vi "TLB Native Dynamic Events ver 0.26b.vi"() -> ()   [LabVIEW 2018] (continued)
                      n634 = Enqueue Element(queue=w1888, element=w1886) -> (queue out=w1887:refnum<queue>)  [unwired: 2 in, 2 out]
                    }
                  }
                }
                n635 = Or(x=w1870, y=w1866) -> (x .or. y?=w1873:bool)
                n636 = Select(t=State_Type_Definitions,_for_0.26g_versions_and_later_2."True Stop" ("Enum"), s=w1866, f=State_Type_Definitions,_for_0.26g_versions_and_later_2."Task 8K: RAISE MY SWORD" ("Enum")) -> (s? t:f=w1868:T18)
                n637 = Select(t=w1868, s=w1873, f=State_Type_Definitions,_for_0.26g_versions_and_later_2."Task 8J: CLOSE CLAW" ("Enum")) -> (s? t:f=w1872:T18)
              }
              frame "Exit" {
                n638 = for {
                  shift-right: [w1895] -> w1892
                  shift-left: w1889 -> [w1896]
                  tunnel: string[] ["STOP", "RESET ENCODERS", "RESET YAW", "ARDUINO MODE 0"] -> [w1894] mode=indexing
                  n639 = Enqueue Element(queue=w1896, element=w1894) -> (queue out=w1895:refnum<queue>)  [unwired: 2 in, 2 out]
                }
              }
            }
          }
          frame 37 {
            # ">>> yStepper command>>>"
            # ">> Manual override >>"
            n640 = Dequeue Element(queue=w1907, timeout in ms (-1)=w1906, error in (no error)=w1908) -> (element=w1905:T10)  [unwired: 3 out]
            n641 = Equal?(x=w1904, y=u8 60) -> (x = y?=w1902:bool)
            n642 = case shown="\"Start Task 1\", Default" w1905 {
              tunnel: [w1918 State_Type_Definitions,_for_0.26g_versions_and_later_2."True Stop" ("Enum")] -> w1909
              tunnel: [w1921 w1938] -> w1910
              tunnel: [State_Type_Definitions,_for_0.26g_versions_and_later_2."Idle" ("Enum") State_Type_Definitions,_for_0.26g_versions_and_later_2."Shutdown" ("Enum")] -> w1911
              tunnel: w1902 -> [w1917 _]
              tunnel: w1901 -> [w1916 _]
              tunnel: w1900 -> [w1912 w1935]
              frame "Start Task 1", Default {
                # "Stays in Task 5_A until stepper reaches desired \nheight"
                # "T: Go back to idle, F: Continue with task\""
                # ">> Manual override >>"
                n643 = case shown="True" w1917 {
                  tunnel: [w1925 w1931] -> w1921
                  tunnel: w1912 -> [w1923 w1929]
                  frame False {
                    n644 = for {
                      tunnel: string[] ["Z STEPPER CAM HEIGHT", "READ STEPPER VALUES"] ("element") -> [w1926] mode=indexing
                      shift-right: [w1928] -> w1925
                      shift-left: w1923 -> [w1927]
                      n645 = Enqueue Element(queue=w1927, element=w1926) -> (queue out=w1928:refnum<queue>)  [unwired: 2 in, 2 out]
                    }
                  }
                  frame True {
                    n646 = for {
                      shift-right: [w1933] -> w1931
                      shift-left: w1929 -> [w1934]
                      tunnel: string[] ["CAM CLOSE", "DISPOSE CAM BUFFERS", "DISPOSE PROC BUFFERS", "RESET ENCODERS"] -> [w1932] mode=indexing
                      n647 = Enqueue Element(queue=w1934, element=w1932) -> (queue out=w1933:refnum<queue>)  [unwired: 2 in, 2 out]
                    }
                  }
                }
                n648 = Or(x=w1917, y=w1916) -> (x .or. y?=w1919:bool)
                n649 = Select(t=State_Type_Definitions,_for_0.26g_versions_and_later_2."True Stop" ("Enum"), s=w1916, f=State_Type_Definitions,_for_0.26g_versions_and_later_2."True Stop" ("Enum")) -> (s? t:f=w1913:T18)
                n650 = Select(t=w1913, s=w1919, f=State_Type_Definitions,_for_0.26g_versions_and_later_2."Task 8K: RAISE MY SWORD" ("Enum")) -> (s? t:f=w1918:T18)
              }
              frame "Exit" {
                n651 = for {
                  shift-right: [w1941] -> w1938
                  shift-left: w1935 -> [w1942]
                  tunnel: string[] ["STOP", "RESET ENCODERS", "RESET YAW", "ARDUINO MODE 0"] -> [w1940] mode=indexing
                  n652 = Enqueue Element(queue=w1942, element=w1940) -> (queue out=w1941:refnum<queue>)  [unwired: 2 in, 2 out]
                }
              }
            }
          }
          frame 38 {
            # ">>> Motor control cluster >>>"
            # ">> Stepper height reeached >>"
            # ">>> yStepper command>>>"
            # ">> Manual override >>"
            n653 = Dequeue Element(queue=w1954, timeout in ms (-1)=w1949, error in (no error)=w1953) -> (element=w1957:T10)  [unwired: 3 out]
            n654 = Equal?(x=w1951, y=u8 50) -> (x = y?=w1955:bool)
            n655 = case shown="\"Start Task 1\", Default" w1957 {
              tunnel: [w1968 State_Type_Definitions,_for_0.26g_versions_and_later_2."True Stop" ("Enum")] -> w1947
              tunnel: [w1966 w1983] -> w1946
              tunnel: w1950 -> [w1965 _]
              tunnel: w1952 -> [w1959 _]
              tunnel: [State_Type_Definitions,_for_0.26g_versions_and_later_2."Idle" ("Enum") State_Type_Definitions,_for_0.26g_versions_and_later_2."Shutdown" ("Enum")] -> w1948
              tunnel: w1955 -> [w1958 _]
              frame "Start Task 1", Default {
                # ">> WIill proceed to part ii if not manual override >>"
                # ">>If ENABLE or Trigger is set to true>>"
                n656 = Or(x=w1958, y=w1959) -> (x .or. y?=w1960:bool)
                n657 = case shown="False" w1958 {
                  tunnel: [w1971 w1977] -> w1966
                  tunnel: w1965 -> [w1970 w1976]
                  frame False {
                    n658 = for {
                      shift-right: [w1973] -> w1971
                      shift-left: w1970 -> [w1974]
                      tunnel: string[] ["Z STEPPER BOX HEIGHT", "READ STEPPER VALUES"] ("element") -> [w1972] mode=indexing
                      n659 = Enqueue Element(queue=w1974, element=w1972) -> (queue out=w1973:refnum<queue>)  [unwired: 2 in, 2 out]
                    }
                  }
                  frame True {
                    n660 = for {
                      shift-right: [w1979] -> w1977
                      shift-left: w1976 -> [w1980]
                      tunnel: string[] ["ARDUINO - ULTRASONIC", "READ NAVX", "RESET FLAGS", "", "", ""] -> [w1978] mode=indexing
                      n661 = Enqueue Element(queue=w1980, element=w1978) -> (queue out=w1979:refnum<queue>)  [unwired: 2 in, 2 out]
                    }
                  }
                }
                n662 = Select(t=State_Type_Definitions,_for_0.26g_versions_and_later_2."True Stop" ("Enum"), s=w1959, f=State_Type_Definitions,_for_0.26g_versions_and_later_2."Task 9B: Rotate to Angle" ("Enum")) -> (s? t:f=w1962:T18)
                n663 = Select(t=w1962, s=w1960, f=State_Type_Definitions,_for_0.26g_versions_and_later_2."Task 9A: Raise Arm" ("Enum")) -> (s? t:f=w1968:T18)
              }
              frame "Exit" {
                n664 = for {
                  shift-right: [w1986] -> w1983
                  shift-left: _ -> [w1987]
                  tunnel: string[] ["STOP", "RESET ENCODERS", "RESET YAW", ""] -> [w1985] mode=indexing
                  n665 = Enqueue Element(queue=w1987, element=w1985) -> (queue out=w1986:refnum<queue>)  [unwired: 2 in, 2 out]
                }
              }
            }
          }
          frame 39 {
            # ">>> Motor control cluster >>>"
            # ">>> yStepper command>>>"
            n666 = Dequeue Element(queue=w2001, timeout in ms (-1)=w2000, error in (no error)=w1999) -> (element=w2003:T10)  [unwired: 3 out]
            n667 = In Range and Coerce(upper limit=65.0, x=w1993, lower limit=58.0) -> (In Range?=w1990:bool)  [unwired: 1 out]
            n668 = case shown="\"Start Task 1\", Default" w2003 {
              tunnel: w1994 -> [w2006 _]
              tunnel: [w2014 State_Type_Definitions,_for_0.26g_versions_and_later_2."True Stop" ("Enum")] -> w1996
              tunnel: w2002 -> [w2012 w2030]
              tunnel: [w2011 w2029] -> w1995
              tunnel: [State_Type_Definitions,_for_0.26g_versions_and_later_2."Idle" ("Enum") State_Type_Definitions,_for_0.26g_versions_and_later_2."Shutdown" ("Enum")] -> w1997
              tunnel: w1990 -> [w2004 _]
              frame "Start Task 1", Default {
                n669 = Or(x=w2004, y=w2006) -> (x .or. y?=w2005:bool)
                n670 = case shown="True" w2004 {
                  tunnel: w2012 -> [w2017 w2023]
                  tunnel: [w2016 w2021] -> w2011
                  frame False {
                    n671 = for {
                      shift-right: [w2019] -> w2016
                      shift-left: w2017 -> [w2020]
                      tunnel: string[] ["READ NAVX", "R-CW", "READ ULTRASONIC"] ("element") -> [w2018] mode=indexing
                      n672 = Enqueue Element(queue=w2020, element=w2018) -> (queue out=w2019:refnum<queue>)  [unwired: 2 in, 2 out]
                    }
                  }
                  frame True {
                    n673 = for {
                      shift-right: [w2025] -> w2021
                      shift-left: w2023 -> [w2026]
                      tunnel: string[] ["STOP", "RESET ENCODERS", "RESET YAW", "ARDUINO - ULTRASONIC", ""] -> [w2024] mode=indexing
                      n674 = Enqueue Element(queue=w2026, element=w2024) -> (queue out=w2025:refnum<queue>)  [unwired: 2 in, 2 out]
                    }
                  }
                }
                n675 = Select(t=State_Type_Definitions,_for_0.26g_versions_and_later_2."True Stop" ("Enum"), s=w2006, f=State_Type_Definitions,_for_0.26g_versions_and_later_2."Task 9C: Detect Box") -> (s? t:f=w2008:T18)
                n676 = Select(t=w2008, s=w2005, f=State_Type_Definitions,_for_0.26g_versions_and_later_2."Task 9B: Rotate to Angle" ("Enum")) -> (s? t:f=w2014:T18)
              }
              frame "Exit" {
                n677 = for {
                  shift-right: [w2033] -> w2029
                  shift-left: w2030 -> [w2034]
                  tunnel: string[] ["STOP", "RESET ENCODERS", "RESET YAW", ""] -> [w2032] mode=indexing
                  n678 = Enqueue Element(queue=w2034, element=w2032) -> (queue out=w2033:refnum<queue>)  [unwired: 2 in, 2 out]
                }
              }
            }
          }
          frame 40 {
            # ">>> Motor control cluster >>>"
            # ">>Line Detected>>"
            # ">>Action Queue>>"
            # ">>> yStepper command>>>"
            n679 = Dequeue Element(queue=w2046, timeout in ms (-1)=w2045, error in (no error)=w2044) -> (element=w2047:T10)  [unwired: 3 out]
            n680 = case shown="\"Start Task 1\", Default" w2047 {
              tunnel: w2042 -> [w2048 _]
              tunnel: [w2058 State_Type_Definitions,_for_0.26g_versions_and_later_2."True Stop" ("Enum")] -> w2039
              tunnel: w2043 -> [w2056 w2074]
              tunnel: [w2055 w2073] -> w2038
              tunnel: [State_Type_Definitions,_for_0.26g_versions_and_later_2."Idle" ("Enum") State_Type_Definitions,_for_0.26g_versions_and_later_2."Shutdown" ("Enum")] -> w2041
              tunnel: w2036 -> [w2049 _]
              frame "Start Task 1", Default {
                n681 = Or(x=w2048, y=w2049) -> (x .or. y?=w2050:bool)
                n682 = case shown="True" w2049 {
                  tunnel: w2056 -> [w2061 w2067]
                  tunnel: [w2060 w2065] -> w2055
                  frame False {
                    n683 = for {
                      shift-right: [w2063] -> w2060
                      shift-left: w2061 -> [w2064]
                      tunnel: string[] ["READ IR", "READ LINE SENSOR", "FORWARD - IR ASSIST"] ("element") -> [w2062] mode=indexing
                      n684 = Enqueue Element(queue=w2064, element=w2062) -> (queue out=w2063:refnum<queue>)  [unwired: 2 in, 2 out]
                    }
                  }
                  frame True {
                    n685 = for {
                      shift-right: [w2069] -> w2065
                      shift-left: w2067 -> [w2070]
                      tunnel: string[] ["STOP", "RESET ENCODERS", "RESET YAW", ""] -> [w2068] mode=indexing
                      n686 = Enqueue Element(queue=w2070, element=w2068) -> (queue out=w2069:refnum<queue>)  [unwired: 2 in, 2 out]
                    }
                  }
                }
                n687 = Select(t=State_Type_Definitions,_for_0.26g_versions_and_later_2."True Stop" ("Enum"), s=w2048, f=State_Type_Definitions,_for_0.26g_versions_and_later_2."Task 9D: MOVE FORWARD") -> (s? t:f=w2052:T18)
                n688 = Select(t=w2052, s=w2050, f=State_Type_Definitions,_for_0.26g_versions_and_later_2."Task 9C: Detect Box" ("Enum")) -> (s? t:f=w2058:T18)
              }
              frame "Exit" {
                n689 = for {
                  shift-right: [w2077] -> w2073
                  shift-left: w2074 -> [w2078]
                  tunnel: string[] ["STOP", "RESET ENCODERS", "RESET YAW", ""] -> [w2076] mode=indexing
                  n690 = Enqueue Element(queue=w2078, element=w2076) -> (queue out=w2077:refnum<queue>)  [unwired: 2 in, 2 out]
                }
              }
            }
          }
          frame 41 {
            (unwired) 50.0 ("y")
            # ">> Item Selection Bias >>"
            # ">> Wall detected >>"
            # ">> Manual override >>"
            # ">>Table Detected>>"
            # ">>> Motor control cluster >>>"
            # ">>Table or wall detectected>>"
            # ">>Action Queue>>"
            # ">>> yStepper command>>>"
            n691 = Dequeue Element(queue=w2096, timeout in ms (-1)=w2095, error in (no error)=w2094) -> (element=w2097:T10)  [unwired: 3 out]
            n692 = Less Or Equal?(x=w2085, y=20.0) -> (x <= y?=w2080:bool)
            n693 = Less?(x=w2083, y=20.0) -> (x < y?=w2081:bool)
            n694 = Or(x=w2080, y=w2081) -> (x .or. y?=w2079:bool)
            n695 = case shown="\"Start Task 1\", Default" w2097 {
              tunnel: w2092 -> [w2098 _]
              tunnel: [w2108 State_Type_Definitions,_for_0.26g_versions_and_later_2."True Stop" ("Enum")] -> w2089
              tunnel: w2093 -> [w2106 w2124]
              tunnel: [w2105 w2123] -> w2088
              tunnel: [State_Type_Definitions,_for_0.26g_versions_and_later_2."Idle" ("Enum") State_Type_Definitions,_for_0.26g_versions_and_later_2."Shutdown" ("Enum")] -> w2091
              tunnel: w2079 -> [w2099 _]
              frame "Start Task 1", Default {
                n696 = Or(x=w2098, y=w2099) -> (x .or. y?=w2100:bool)
                n697 = case shown="False" w2099 {
                  tunnel: w2106 -> [w2111 w2117]
                  tunnel: [w2110 w2115] -> w2105
                  frame False {
                    n698 = for {
                      shift-right: [w2113] -> w2110
                      shift-left: w2111 -> [w2114]
                      tunnel: string[] ["READ IR", "FORWARD - IR ASSIST", "READ ULTRASONIC"] ("element") -> [w2112] mode=indexing
                      n699 = Enqueue Element(queue=w2114, element=w2112) -> (queue out=w2113:refnum<queue>)  [unwired: 2 in, 2 out]
                    }
                  }
                  frame True {
                    n700 = for {
                      shift-right: [w2119] -> w2115
                      shift-left: w2117 -> [w2120]
                      tunnel: string[] ["STOP", "RESET ENCODERS", "RESET YAW", ""] -> [w2118] mode=indexing
                      n701 = Enqueue Element(queue=w2120, element=w2118) -> (queue out=w2119:refnum<queue>)  [unwired: 2 in, 2 out]
                    }
                  }
                }
                n702 = Select(t=State_Type_Definitions,_for_0.26g_versions_and_later_2."True Stop" ("Enum"), s=w2098, f=State_Type_Definitions,_for_0.26g_versions_and_later_2."Task 9E: MOVE LEFT") -> (s? t:f=w2102:T18)
                n703 = Select(t=w2102, s=w2100, f=State_Type_Definitions,_for_0.26g_versions_and_later_2."Task 9D: MOVE FORWARD" ("Enum")) -> (s? t:f=w2108:T18)
              }
              frame "Exit" {
                n704 = for {
                  shift-right: [w2127] -> w2123
                  shift-left: w2124 -> [w2128]
                  tunnel: string[] ["STOP", "RESET ENCODERS", "RESET YAW", ""] -> [w2126] mode=indexing
                  n705 = Enqueue Element(queue=w2128, element=w2126) -> (queue out=w2127:refnum<queue>)  [unwired: 2 in, 2 out]
                }
              }
            }
          }
          frame 42 {
            # ">> Item Selection Bias >>"
            # ">> Line detected? >>"
            # ">> Manual override >>"
            # ">>> Motor control cluster >>>"
            # ">>Action Queue>>"
            # ">>> yStepper command>>>"
            n706 = Dequeue Element(queue=w2140, timeout in ms (-1)=w2139, error in (no error)=w2138) -> (element=w2141:T10)  [unwired: 3 out]
            n707 = case shown="\"Start Task 1\", Default" w2141 {
              tunnel: w2136 -> [w2142 _]
              tunnel: [w2152 State_Type_Definitions,_for_0.26g_versions_and_later_2."True Stop" ("Enum")] -> w2133
              tunnel: w2137 -> [w2150 w2168]
              tunnel: [w2149 w2167] -> w2132
              tunnel: [State_Type_Definitions,_for_0.26g_versions_and_later_2."Idle" ("Enum") State_Type_Definitions,_for_0.26g_versions_and_later_2."Shutdown" ("Enum")] -> w2135
              tunnel: w2129 -> [w2143 _]
              frame "Start Task 1", Default {
                n708 = Or(x=w2142, y=w2143) -> (x .or. y?=w2144:bool)
                n709 = case shown="False" w2143 {
                  tunnel: w2150 -> [w2155 w2161]
                  tunnel: [w2154 w2159] -> w2149
                  frame False {
                    n710 = for {
                      shift-right: [w2157] -> w2154
                      shift-left: w2155 -> [w2158]
                      tunnel: string[] ["LEFT", "READ NAVX", "READ LINE SENSOR", ""] ("element") -> [w2156] mode=indexing
                      n711 = Enqueue Element(queue=w2158, element=w2156) -> (queue out=w2157:refnum<queue>)  [unwired: 2 in, 2 out]
                    }
                  }
                  frame True {
                    n712 = for {
                      shift-right: [w2163] -> w2159
                      shift-left: w2161 -> [w2164]
                      tunnel: string[] ["STOP", "RESET ENCODERS", "RESET YAW", "RESET FLAGS", "OPEN LIFE CAM", "SET TIMER 2"] -> [w2162] mode=indexing
                      n713 = Enqueue Element(queue=w2164, element=w2162) -> (queue out=w2163:refnum<queue>)  [unwired: 2 in, 2 out]
                    }
                  }
                }
                n714 = Select(t=State_Type_Definitions,_for_0.26g_versions_and_later_2."True Stop" ("Enum"), s=w2142, f=State_Type_Definitions."Task 9F: SCAN IMAGE") -> (s? t:f=w2146:u16)
                n715 = Select(t=w2146, s=w2144, f=State_Type_Definitions,_for_0.26g_versions_and_later_2."Task 9E: MOVE LEFT" ("Enum")) -> (s? t:f=w2152:u16)
              }
              frame "Exit" {
                n716 = for {
                  shift-right: [w2171] -> w2167
                  shift-left: w2168 -> [w2172]
                  tunnel: string[] ["STOP", "RESET ENCODERS", "RESET YAW", ""] -> [w2170] mode=indexing
                  n717 = Enqueue Element(queue=w2172, element=w2170) -> (queue out=w2171:refnum<queue>)  [unwired: 2 in, 2 out]
                }
              }
            }
          }
          frame 43 {
            # ">>> Motor control cluster >>>"
            # ">>Time up? >>"
            # ">>> yStepper command>>>"
            # ">> Manual override >>"
            n718 = Dequeue Element(queue=w2184, timeout in ms (-1)=w2180, error in (no error)=w2183) -> (element=w2185:T10)  [unwired: 3 out]
            n719 = case shown="\"Start Task 1\", Default" w2185 {
              tunnel: [w2196 State_Type_Definitions,_for_0.26g_versions_and_later_2."True Stop" ("Enum")] -> w2178
              tunnel: [w2194 w2212] -> w2177
              tunnel: w2181 -> [w2193 w2209]
              tunnel: w2182 -> [w2187 _]
              tunnel: [State_Type_Definitions,_for_0.26g_versions_and_later_2."Idle" ("Enum") State_Type_Definitions,_for_0.26g_versions_and_later_2."Shutdown" ("Enum")] -> w2179
              tunnel: w2173 -> [w2186 _]
              frame "Start Task 1", Default {
                # ">> WIill proceed to part ii if not manual override >>"
                # ">>If ENABLE or Trigger is set to true>>"
                n720 = Or(x=w2186, y=w2187) -> (x .or. y?=w2188:bool)
                n721 = case shown="True" w2186 {
                  tunnel: [w2199 w2205] -> w2194
                  tunnel: w2193 -> [w2198 w2204]
                  frame False {
                    n722 = for {
                      shift-right: [w2201] -> w2199
                      shift-left: w2198 -> [w2202]
                      tunnel: string[] ["CAM ACQ", "START TIMER"] ("element") -> [w2200] mode=indexing
                      n723 = Enqueue Element(queue=w2202, element=w2200) -> (queue out=w2201:refnum<queue>)  [unwired: 2 in, 2 out]
                    }
                  }
                  frame True {
                    n724 = for {
                      shift-right: [w2207] -> w2205
                      shift-left: w2204 -> [w2208]
                      tunnel: string[] ["CLOSE CAM", "SET TIMER 5", "", "", "", ""] -> [w2206] mode=indexing
                      n725 = Enqueue Element(queue=w2208, element=w2206) -> (queue out=w2207:refnum<queue>)  [unwired: 2 in, 2 out]
                    }
                  }
                }
                n726 = Select(t=State_Type_Definitions,_for_0.26g_versions_and_later_2."True Stop" ("Enum"), s=w2187, f=State_Type_Definitions."Task 9G: PROCESS COLOUR" ("Enum")) -> (s? t:f=w2190:u16)
                n727 = Select(t=w2190, s=w2188, f=State_Type_Definitions."Task 9F: SCAN IMAGE" ("Enum")) -> (s? t:f=w2196:u16)
              }
              frame "Exit" {
                n728 = for {
                  shift-right: [w2215] -> w2212
                  shift-left: w2209 -> [w2216]
                  tunnel: string[] ["STOP", "RESET ENCODERS", "RESET YAW", ""] -> [w2214] mode=indexing
                  n729 = Enqueue Element(queue=w2216, element=w2214) -> (queue out=w2215:refnum<queue>)  [unwired: 2 in, 2 out]
                }
              }
            }
          }
          frame 44 {
            # ">>> Motor control cluster >>>"
            # ">>> yStepper command>>>"
            n730 = Dequeue Element(queue=w2224, timeout in ms (-1)=w2223, error in (no error)=w2222) -> (element=w2229:T10)  [unwired: 3 out]
            n731 = case shown="\"Start Task 1\", Default" w2229 {
              tunnel: w2217 -> [w2232 _]
              tunnel: [w2239 State_Type_Definitions,_for_0.26g_versions_and_later_2."True Stop" ("Enum")] -> w2228
              tunnel: w2221 -> [w2231 _]
              tunnel: w2225 -> [w2238 w2255]
              tunnel: [w2237 w2256] -> w2227
              tunnel: [State_Type_Definitions,_for_0.26g_versions_and_later_2."Idle" ("Enum") State_Type_Definitions,_for_0.26g_versions_and_later_2."Shutdown" ("Enum")] -> w2226
              frame "Start Task 1", Default {
                n732 = case shown="False" w2232 {
                  tunnel: w2238 -> [w2242 w2249]
                  tunnel: [w2243 w2248] -> w2237
                  frame False {
                    n733 = for {
                      tunnel: string[] ["START TIMER", "COLOUR PROCESSING", ""] ("element") -> [w2244] mode=indexing
                      shift-right: [w2246] -> w2243
                      shift-left: w2242 -> [w2245]
                      n734 = Enqueue Element(queue=w2245, element=w2244) -> (queue out=w2246:refnum<queue>)  [unwired: 2 in, 2 out]
                    }
                  }
                  frame True {
                    n735 = for {
                      shift-right: [w2251] -> w2248
                      shift-left: w2249 -> [w2252]
                      tunnel: string[] ["DISPOSE BUFFERS", "CLOSE CAM", "RESET ENCODERS", "RESET YAW", "RESET FLAGS"] -> [w2250] mode=indexing
                      n736 = Enqueue Element(queue=w2252, element=w2250) -> (queue out=w2251:refnum<queue>)  [unwired: 2 in, 2 out]
                    }
                  }
                }
                n737 = Or(x=w2232, y=w2231) -> (x .or. y?=w2230:bool)
                n738 = Select(t=State_Type_Definitions,_for_0.26g_versions_and_later_2."True Stop" ("Enum"), s=w2231, f=State_Type_Definitions."Task 9G: PROCESS COLOUR" ("Enum")) -> (s? t:f=w2233:u16)
                n739 = Select(t=w2233, s=w2230, f=State_Type_Definitions."Task 9G: PROCESS COLOUR" ("Enum")) -> (s? t:f=w2239:u16)
              }
              frame "Exit" {
                n740 = for {
                  shift-right: [w2259] -> w2256
                  shift-left: w2255 -> [w2260]
                  tunnel: string[] ["STOP", "RESET ENCODERS", "RESET YAW", "ARDUINO MODE 0"] -> [w2258] mode=indexing
                  n741 = Enqueue Element(queue=w2260, element=w2258) -> (queue out=w2259:refnum<queue>)  [unwired: 2 in, 2 out]
                }
              }
            }
          }
          frame 45 {
            # ">> Item Selection Bias >>"
            # ">>> Motor control cluster >>>"
            # ">>> yStepper command>>>"
            n742 = Dequeue Element(queue=w2270, timeout in ms (-1)=w2271, error in (no error)=w2272) -> (element=w2274:T10)  [unwired: 3 out]
            n743 = Greater?(x=w2262, y=50.0) -> (0:w2263:bool)
            n744 = And(x=w2264, y=w2263) -> (x .and. y?=w2265:bool)
            n745 = case shown="\"Start Task 1\", Default" w2274 {
              tunnel: w2265 -> [w2280 _]
              tunnel: [w2287 State_Type_Definitions,_for_0.26g_versions_and_later_2."True Stop" ("Enum")] -> w2267
              tunnel: w2273 -> [w2279 _]
              tunnel: w2269 -> [w2286 w2303]
              tunnel: [w2285 w2304] -> w2268
              tunnel: [State_Type_Definitions,_for_0.26g_versions_and_later_2."Idle" ("Enum") State_Type_Definitions,_for_0.26g_versions_and_later_2."Shutdown" ("Enum")] -> w2266
              frame "Start Task 1", Default {
                n746 = case shown="True" w2280 {
                  tunnel: w2286 -> [w2290 w2297]
                  tunnel: [w2291 w2296] -> w2285
                  frame False {
                    n747 = for {
                      tunnel: string[] ["READ LINE SENSOR", "READ NAVX", "RIGHT", "READ ENCODERS"] ("element") -> [w2292] mode=indexing
                      shift-right: [w2294] -> w2291
                      shift-left: w2290 -> [w2293]
                      n748 = Enqueue Element(queue=w2293, element=w2292) -> (queue out=w2294:refnum<queue>)  [unwired: 2 in, 2 out]
                    }
                  }
                  frame True {
                    n749 = for {
                      shift-right: [w2299] -> w2296
                      shift-left: w2297 -> [w2300]
                      tunnel: string[] ["STOP", "RESET ENCODERS", "RESET YAW", "OPEN LIFE CAM", "SET TIMER 5", "RESET FLAGS"] -> [w2298] mode=indexing
                      n750 = Enqueue Element(queue=w2300, element=w2298) -> (queue out=w2299:refnum<queue>)  [unwired: 2 in, 2 out]
                    }
                  }
                }
                n751 = Or(x=w2280, y=w2279) -> (x .or. y?=w2278:bool)
                n752 = Select(t=State_Type_Definitions,_for_0.26g_versions_and_later_2."True Stop" ("Enum"), s=w2279, f=State_Type_Definitions,_for_0.26d_versions_and_later."Task 9I: SCAN IMAGE" ("Enum")) -> (s? t:f=w2281:u16)
                n753 = Select(t=w2281, s=w2278, f=State_Type_Definitions."Task 9H: MOVE RIGHT" ("Enum")) -> (s? t:f=w2287:u16)
              }
              frame "Exit" {
                n754 = for {
                  shift-right: [w2307] -> w2304
                  shift-left: w2303 -> [w2308]
                  tunnel: string[] ["STOP", "RESET ENCODERS", "RESET YAW", "ARDUINO MODE 0"] -> [w2306] mode=indexing
                  n755 = Enqueue Element(queue=w2308, element=w2306) -> (queue out=w2307:refnum<queue>)  [unwired: 2 in, 2 out]
                }
              }
            }
          }
          frame 46 {
            # ">> Item Selection Bias >>"
            n756 = Dequeue Element(queue=w2310, timeout in ms (-1)=w2311, error in (no error)=w2312) -> (element=w2318:T10)  [unwired: 3 out]
            n757 = case shown="\"Start Task 1\", Default" w2318 {
              tunnel: w2309 -> [w2324 _]
              tunnel: [w2331 State_Type_Definitions,_for_0.26g_versions_and_later_2."True Stop" ("Enum")] -> w2315
              tunnel: w2313 -> [w2323 _]
              tunnel: w2317 -> [w2330 w2347]
              tunnel: [w2329 w2348] -> w2316
              tunnel: [State_Type_Definitions,_for_0.26g_versions_and_later_2."Idle" ("Enum") State_Type_Definitions,_for_0.26g_versions_and_later_2."Shutdown" ("Enum")] -> w2314
              frame "Start Task 1", Default {
                n758 = case shown="True" w2324 {
                  tunnel: w2330 -> [w2334 w2341]
                  tunnel: [w2335 w2340] -> w2329
                  frame False {
                    n759 = for {
                      tunnel: string[] ["START TIMER", "CAM ACQ", ""] ("element") -> [w2336] mode=indexing
                      shift-right: [w2338] -> w2335
                      shift-left: w2334 -> [w2337]
                      n760 = Enqueue Element(queue=w2337, element=w2336) -> (queue out=w2338:refnum<queue>)  [unwired: 2 in, 2 out]
                    }
                  }
                  frame True {
                    n761 = for {
                      shift-right: [w2343] -> w2340
                      shift-left: w2341 -> [w2344]
                      tunnel: string[] ["CLOSE CAM", "SET TIMER 5", "", "", "", ""] -> [w2342] mode=indexing
                      n762 = Enqueue Element(queue=w2344, element=w2342) -> (queue out=w2343:refnum<queue>)  [unwired: 2 in, 2 out]
                    }
                  }
                }
                n763 = Or(x=w2324, y=w2323) -> (x .or. y?=w2322:bool)
                n764 = Select(t=State_Type_Definitions,_for_0.26g_versions_and_later_2."True Stop" ("Enum"), s=w2323, f=State_Type_Definitions,_for_0.26d_versions_and_later."Task 9J: PROCESS COLOUR" ("Enum")) -> (s? t:f=w2325:u16)
                n765 = Select(t=w2325, s=w2322, f=State_Type_Definitions,_for_0.26d_versions_and_later."Task 9I: SCAN IMAGE" ("Enum")) -> (s? t:f=w2331:u16)
              }
              frame "Exit" {
                n766 = for {
                  shift-right: [w2351] -> w2348
                  shift-left: w2347 -> [w2352]
                  tunnel: string[] ["STOP", "RESET ENCODERS", "RESET YAW", "ARDUINO MODE 0"] -> [w2350] mode=indexing
                  n767 = Enqueue Element(queue=w2352, element=w2350) -> (queue out=w2351:refnum<queue>)  [unwired: 2 in, 2 out]
                }
              }
            }
          }
          frame 47 {
            # ">> Item Selection Bias >>"
            n768 = Dequeue Element(queue=w2358, timeout in ms (-1)=w2359, error in (no error)=w2360) -> (element=w2362:T10)  [unwired: 3 out]
            n769 = case shown="\"Start Task 1\", Default" w2362 {
              tunnel: w2353 -> [w2368 _]
              tunnel: [w2375 State_Type_Definitions,_for_0.26g_versions_and_later_2."True Stop" ("Enum")] -> w2356
              tunnel: w2361 -> [w2367 _]
              tunnel: w2357 -> [w2374 w2391]
              tunnel: [w2373 w2392] -> w2355
              tunnel: [State_Type_Definitions,_for_0.26g_versions_and_later_2."Idle" ("Enum") State_Type_Definitions,_for_0.26g_versions_and_later_2."Shutdown" ("Enum")] -> w2354
              frame "Start Task 1", Default {
                n770 = case shown="True" w2368 {
                  tunnel: w2374 -> [w2378 w2385]
                  tunnel: [w2379 w2384] -> w2373
                  frame False {
                    n771 = for {
                      tunnel: string[] ["START TIMER", "COLOUR PROCESSING", ""] ("element") -> [w2380] mode=indexing
                      shift-right: [w2382] -> w2379
                      shift-left: w2378 -> [w2381]
                      n772 = Enqueue Element(queue=w2381, element=w2380) -> (queue out=w2382:refnum<queue>)  [unwired: 2 in, 2 out]
                    }
                  }
                  frame True {
                    n773 = for {
                      shift-right: [w2387] -> w2384
                      shift-left: w2385 -> [w2388]
                      tunnel: string[] ["CLOSE CAM", "DISPOSE BUFFERS", "RESET ENCODERS", "RESET YAW", "RESET FLAGS", ""] -> [w2386] mode=indexing
                      n774 = Enqueue Element(queue=w2388, element=w2386) -> (queue out=w2387:refnum<queue>)  [unwired: 2 in, 2 out]
                    }
                  }
                }
                n775 = Or(x=w2368, y=w2367) -> (x .or. y?=w2366:bool)
                n776 = Select(t=State_Type_Definitions,_for_0.26g_versions_and_later_2."True Stop" ("Enum"), s=w2367, f=State_Type_Definitions,_for_0.26g_versions_and_later_2."True Stop" ("Enum")) -> (s? t:f=w2369:T18)
                n777 = Select(t=w2369, s=w2366, f=State_Type_Definitions,_for_0.26d_versions_and_later."Task 9J: PROCESS COLOUR" ("Enum")) -> (s? t:f=w2375:u16)
              }
              frame "Exit" {
                n778 = for {
                  shift-right: [w2395] -> w2392
                  shift-left: w2391 -> [w2396]
                  tunnel: string[] ["STOP", "RESET ENCODERS", "RESET YAW", "ARDUINO MODE 0"] -> [w2394] mode=indexing
                  n779 = Enqueue Element(queue=w2396, element=w2394) -> (queue out=w2395:refnum<queue>)  [unwired: 2 in, 2 out]
                }
              }
            }
          }
          frame 48 {
            # ">>> Motor control cluster >>>"
            # ">>> yStepper command>>>"
            # ">> Item Selection Bias >>"
            n780 = Less?(x=w2400, y=-38.0) -> (x < y?=w2398:bool)
            n781 = Dequeue Element(queue=w2406, timeout in ms (-1)=w2405, error in (no error)=w2404) -> (element=w2408:T10)  [unwired: 3 out]
            n782 = case shown="\"Start Task 1\", Default" w2408 {
              tunnel: w2398 -> [w2414 _]
              tunnel: [w2421 State_Type_Definitions,_for_0.26g_versions_and_later_2."True Stop" ("Enum")] -> w2402
              tunnel: w2403 -> [w2413 _]
              tunnel: w2407 -> [w2420 w2437]
              tunnel: [w2419 w2438] -> w2397
              tunnel: [State_Type_Definitions,_for_0.26g_versions_and_later_2."Idle" ("Enum") State_Type_Definitions,_for_0.26g_versions_and_later_2."Shutdown" ("Enum")] -> w2401
              frame "Start Task 1", Default {
                n783 = case shown="True" w2414 {
                  tunnel: w2420 -> [w2424 w2431]
                  tunnel: [w2425 w2430] -> w2419
                  frame False {
                    n784 = for {
                      tunnel: string[] ["READ ENCODERS", "R-CW"] ("element") -> [w2426] mode=indexing
                      shift-right: [w2428] -> w2425
                      shift-left: w2424 -> [w2427]
                      n785 = Enqueue Element(queue=w2427, element=w2426) -> (queue out=w2428:refnum<queue>)  [unwired: 2 in, 2 out]
                    }
                  }
                  frame True {
                    n786 = for {
                      shift-right: [w2433] -> w2430
                      shift-left: w2431 -> [w2434]
                      tunnel: string[] ["STOP", "RESET ENCODERS", "RESET FLAGS", "RESET YAW", "READ IR", "ARDUINO - ULTRASONIC"] -> [w2432] mode=indexing
                      n787 = Enqueue Element(queue=w2434, element=w2432) -> (queue out=w2433:refnum<queue>)  [unwired: 2 in, 2 out]
                    }
                  }
                }
                n788 = Or(x=w2414, y=w2413) -> (x .or. y?=w2412:bool)
                n789 = Select(t=State_Type_Definitions,_for_0.26g_versions_and_later_2."True Stop" ("Enum"), s=w2413, f=State_Type_Definitions,_for_0.26d_versions_and_later."Task 9L: MOVE FORWARD" ("Enum")) -> (s? t:f=w2415:u16)
                n790 = Select(t=w2415, s=w2412, f=State_Type_Definitions,_for_0.26d_versions_and_later."Task 9K: ROTATE 90 CW" ("Enum")) -> (s? t:f=w2421:u16)
              }
              frame "Exit" {
                n791 = for {
                  shift-right: [w2441] -> w2438
                  shift-left: w2437 -> [w2442]
                  tunnel: string[] ["STOP", "RESET ENCODERS", "RESET YAW", "ARDUINO MODE 0"] -> [w2440] mode=indexing
                  n792 = Enqueue Element(queue=w2442, element=w2440) -> (queue out=w2441:refnum<queue>)  [unwired: 2 in, 2 out]
                }
              }
            }
          }
          frame 49 {
            w2455 = u8 50 ("y")
            # ">>> Motor control cluster >>>"
            # ">>> yStepper command>>>"
            # ">> Item Selection Bias >>"
            n793 = Less?(x=w2457, y=w2455) -> (x < y?=w2450:bool)
            n794 = Dequeue Element(queue=w2461, timeout in ms (-1)=w2460, error in (no error)=w2459) -> (element=w2465:T10)  [unwired: 3 out]
            n795 = Less?(x=w2456, y=w2455) -> (x < y?=w2451:bool)
            n796 = And(x=w2451, y=w2450) -> (x .and. y?=w2443:bool)
            n797 = Less Or Equal?(x=w2454, y=15.0) -> (x <= y?=w2449:bool)
            n798 = Greater?(x=w2448, y=100.0) -> (0:w2447:bool)
            n799 = Or(x=w2449, y=w2443) -> (x .or. y?=w2445:bool)
            n800 = And(x=w2447, y=w2445) -> (x .and. y?=w2446:bool)
            n801 = case shown="\"Start Task 1\", Default" w2465 {
              tunnel: w2446 -> [w2471 _]
              tunnel: [w2478 State_Type_Definitions,_for_0.26g_versions_and_later_2."True Stop" ("Enum")] -> w2463
              tunnel: w2458 -> [w2470 _]
              tunnel: w2462 -> [w2477 w2494]
              tunnel: [w2476 w2495] -> w2452
              tunnel: [State_Type_Definitions,_for_0.26g_versions_and_later_2."Idle" ("Enum") State_Type_Definitions,_for_0.26g_versions_and_later_2."Shutdown" ("Enum")] -> w2464
              frame "Start Task 1", Default {
                n802 = case shown="True" w2471 {
                  tunnel: w2477 -> [w2481 w2488]
                  tunnel: [w2482 w2487] -> w2476
                  frame False {
                    n803 = for {
                      tunnel: string[] ["READ IR", "FORWARD", "READ NAVX", "READ ENCODERS"] ("element") -> [w2483] mode=indexing
                      shift-right: [w2485] -> w2482
                      shift-left: w2481 -> [w2484]
                      n804 = Enqueue Element(queue=w2484, element=w2483) -> (queue out=w2485:refnum<queue>)  [unwired: 2 in, 2 out]
                    }
                  }
                  frame True {
                    n805 = for {
                      shift-right: [w2490] -> w2487
                      shift-left: w2488 -> [w2491]
                      tunnel: string[] ["STOP", "RESET ENCODERS", "RESET FLAGS", "RESET YAW", "", ""] -> [w2489] mode=indexing
                      n806 = Enqueue Element(queue=w2491, element=w2489) -> (queue out=w2490:refnum<queue>)  [unwired: 2 in, 2 out]
                    }
                  }
                }
                n807 = Or(x=w2471, y=w2470) -> (x .or. y?=w2469:bool)
                n808 = Select(t=State_Type_Definitions,_for_0.26g_versions_and_later_2."True Stop" ("Enum"), s=w2470, f=State_Type_Definitions,_for_0.26g_versions_and_later_2."True Stop" ("Enum")) -> (s? t:f=w2472:T18)
                n809 = Select(t=w2472, s=w2469, f=State_Type_Definitions,_for_0.26d_versions_and_later."Task 9L: MOVE FORWARD" ("Enum")) -> (s? t:f=w2478:u16)
              }
              frame "Exit" {
                n810 = for {
                  shift-right: [w2498] -> w2495
                  shift-left: w2494 -> [w2499]
                  tunnel: string[] ["STOP", "RESET ENCODERS", "RESET YAW", "ARDUINO MODE 0"] -> [w2497] mode=indexing
                  n811 = Enqueue Element(queue=w2499, element=w2497) -> (queue out=w2498:refnum<queue>)  [unwired: 2 in, 2 out]
                }
              }
            }
          }
          frame 50 {
            # ">> Item Selection Bias >>"
            n812 = Dequeue Element(queue=w2504, timeout in ms (-1)=w2503, error in (no error)=w2502) -> (element=w2509:T10)  [unwired: 3 out]
            n813 = case shown="\"Start Task 1\", Default" w2509 {
              tunnel: w2500 -> [w2515 _]
              tunnel: [w2522 State_Type_Definitions,_for_0.26g_versions_and_later_2."True Stop" ("Enum")] -> w2507
              tunnel: w2501 -> [w2514 _]
              tunnel: w2505 -> [w2521 w2538]
              tunnel: [w2520 w2539] -> w2506
              tunnel: [State_Type_Definitions,_for_0.26g_versions_and_later_2."Idle" ("Enum") State_Type_Definitions,_for_0.26g_versions_and_later_2."Shutdown" ("Enum")] -> w2508
              frame "Start Task 1", Default {
                n814 = case shown="False" w2515 {
                  tunnel: w2521 -> [w2525 w2532]
                  tunnel: [w2526 w2531] -> w2520
                  frame False {
                    n815 = for {
                      tunnel: string[] ["READ LINE SENSOR", "READ NAVX", "RIGHT", "READ ENCODERS"] ("element") -> [w2527] mode=indexing
                      shift-right: [w2529] -> w2526
                      shift-left: w2525 -> [w2528]
                      n816 = Enqueue Element(queue=w2528, element=w2527) -> (queue out=w2529:refnum<queue>)  [unwired: 2 in, 2 out]
                    }
                  }
                  frame True {
                    n817 = for {
                      shift-right: [w2534] -> w2531
                      shift-left: w2532 -> [w2535]
                      tunnel: string[] ["STOP", "RESET ENCODERS", "RESET YAW", "OPEN LIFE CAM", "SET TIMER 2", "RESET FLAGS"] -> [w2533] mode=indexing
                      n818 = Enqueue Element(queue=w2535, element=w2533) -> (queue out=w2534:refnum<queue>)  [unwired: 2 in, 2 out]
                    }
                  }
                }
                n819 = Or(x=w2515, y=w2514) -> (x .or. y?=w2513:bool)
                n820 = Select(t=State_Type_Definitions,_for_0.26g_versions_and_later_2."True Stop" ("Enum"), s=w2514, f=State_Type_Definitions,_for_0.26d_versions_and_later."Task 9N: SCAN IMAGE" ("Enum")) -> (s? t:f=w2516:u16)
                n821 = Select(t=w2516, s=w2513, f=State_Type_Definitions,_for_0.26g_versions_and_later_2."Task 9M: MOVE RIGHT" ("Enum")) -> (s? t:f=w2522:u16)
              }
              frame "Exit" {
                n822 = for {
                  shift-right: [w2542] -> w2539
                  shift-left: w2538 -> [w2543]
                  tunnel: string[] ["STOP", "RESET ENCODERS", "RESET YAW", "ARDUINO MODE 0"] -> [w2541] mode=indexing
                  n823 = Enqueue Element(queue=w2543, element=w2541) -> (queue out=w2542:refnum<queue>)  [unwired: 2 in, 2 out]
                }
              }
            }
          }
          frame 51 {
            # ">> Manual override >>"
            n824 = Dequeue Element(queue=w2552, timeout in ms (-1)=w2551, error in (no error)=w2550) -> (element=w2553:T10)  [unwired: 3 out]
            n825 = case shown="\"Start Task 1\", Default" w2553 {
              tunnel: [w2567 State_Type_Definitions,_for_0.26g_versions_and_later_2."True Stop" ("Enum")] -> w2545
              tunnel: [w2565 w2583] -> w2544
              tunnel: w2548 -> [w2564 w2580]
              tunnel: w2549 -> [w2558 _]
              tunnel: [State_Type_Definitions,_for_0.26g_versions_and_later_2."Idle" ("Enum") State_Type_Definitions,_for_0.26g_versions_and_later_2."Shutdown" ("Enum")] -> w2546
              tunnel: w2547 -> [w2557 _]
              frame "Start Task 1", Default {
                # ">> WIill proceed to part ii if not manual override >>"
                # ">>If ENABLE or Trigger is set to true>>"
                n826 = Or(x=w2557, y=w2558) -> (x .or. y?=w2559:bool)
                n827 = case shown="False" w2557 {
                  tunnel: [w2570 w2576] -> w2565
                  tunnel: w2564 -> [w2569 w2575]
                  frame False {
                    n828 = for {
                      shift-right: [w2572] -> w2570
                      shift-left: w2569 -> [w2573]
                      tunnel: string[] ["CAM ACQ", "START TIMER"] ("element") -> [w2571] mode=indexing
                      n829 = Enqueue Element(queue=w2573, element=w2571) -> (queue out=w2572:refnum<queue>)  [unwired: 2 in, 2 out]
                    }
                  }
                  frame True {
                    n830 = for {
                      shift-right: [w2578] -> w2576
                      shift-left: w2575 -> [w2579]
                      tunnel: string[] ["CLOSE CAM", "SET TIMER 5", "", "", "", ""] -> [w2577] mode=indexing
                      n831 = Enqueue Element(queue=w2579, element=w2577) -> (queue out=w2578:refnum<queue>)  [unwired: 2 in, 2 out]
                    }
                  }
                }
                n832 = Select(t=State_Type_Definitions,_for_0.26g_versions_and_later_2."True Stop" ("Enum"), s=w2558, f=State_Type_Definitions,_for_0.26d_versions_and_later."Task 9O: PROCESS COLOUR" ("Enum")) -> (s? t:f=w2561:u16)
                n833 = Select(t=w2561, s=w2559, f=State_Type_Definitions,_for_0.26d_versions_and_later."Task 9N: SCAN IMAGE" ("Enum")) -> (s? t:f=w2567:u16)
              }
              frame "Exit" {
                n834 = for {
                  shift-right: [w2586] -> w2583
                  shift-left: w2580 -> [w2587]
                  tunnel: string[] ["STOP", "RESET ENCODERS", "RESET YAW", ""] -> [w2585] mode=indexing
                  n835 = Enqueue Element(queue=w2587, element=w2585) -> (queue out=w2586:refnum<queue>)  [unwired: 2 in, 2 out]
                }
              }
            }
          }
          frame 52 {
            # ">> Item Selection Bias >>"
            n836 = Dequeue Element(queue=w2595, timeout in ms (-1)=w2594, error in (no error)=w2593) -> (element=w2597:T10)  [unwired: 3 out]
            n837 = case shown="\"Start Task 1\", Default" w2597 {
              tunnel: w2588 -> [w2603 _]
              tunnel: [w2610 State_Type_Definitions,_for_0.26g_versions_and_later_2."True Stop" ("Enum")] -> w2591
              tunnel: w2592 -> [w2602 _]
              tunnel: w2596 -> [w2609 w2626]
              tunnel: [w2608 w2627] -> w2590
              tunnel: [State_Type_Definitions,_for_0.26g_versions_and_later_2."Idle" ("Enum") State_Type_Definitions,_for_0.26g_versions_and_later_2."Shutdown" ("Enum")] -> w2589
              frame "Start Task 1", Default {
                n838 = case shown="False" w2603 {
                  tunnel: w2609 -> [w2613 w2620]
                  tunnel: [w2614 w2619] -> w2608
                  frame False {
                    n839 = for {
                      tunnel: string[] ["START TIMER", "COLOUR PROCESSING", ""] ("element") -> [w2615] mode=indexing
                      shift-right: [w2617] -> w2614
                      shift-left: w2613 -> [w2616]
                      n840 = Enqueue Element(queue=w2616, element=w2615) -> (queue out=w2617:refnum<queue>)  [unwired: 2 in, 2 out]
                    }
                  }
                  frame True {
                    n841 = for {
                      shift-right: [w2622] -> w2619
                      shift-left: w2620 -> [w2623]
                      tunnel: string[] ["CLOSE CAM", "DISPOSE BUFFERS", "RESET ENCODERS", "RESET YAW", "RESET FLAGS", ""] -> [w2621] mode=indexing
                      n842 = Enqueue Element(queue=w2623, element=w2621) -> (queue out=w2622:refnum<queue>)  [unwired: 2 in, 2 out]
                    }
                  }
                }
                n843 = Or(x=w2603, y=w2602) -> (x .or. y?=w2601:bool)
                n844 = Select(t=State_Type_Definitions,_for_0.26g_versions_and_later_2."True Stop" ("Enum"), s=w2602, f=State_Type_Definitions,_for_0.26d_versions_and_later."Task 9P: MOVE RIGHT" ("Enum")) -> (s? t:f=w2604:u16)
                n845 = Select(t=w2604, s=w2601, f=State_Type_Definitions,_for_0.26d_versions_and_later."Task 9O: PROCESS COLOUR" ("Enum")) -> (s? t:f=w2610:u16)
              }
              frame "Exit" {
                n846 = for {
                  shift-right: [w2630] -> w2627
                  shift-left: w2626 -> [w2631]
                  tunnel: string[] ["STOP", "RESET ENCODERS", "RESET YAW", "ARDUINO MODE 0"] -> [w2629] mode=indexing
                  n847 = Enqueue Element(queue=w2631, element=w2629) -> (queue out=w2630:refnum<queue>)  [unwired: 2 in, 2 out]
                }
              }
            }
          }
          frame 53 {
            # ">> Item Selection Bias >>"
            n848 = Dequeue Element(queue=w2637, timeout in ms (-1)=w2636, error in (no error)=w2635) -> (element=w2645:T10)  [unwired: 3 out]
            n849 = Greater?(x=w2633, y=50.0) -> (0:w2643:bool)
            n850 = And(x=w2632, y=w2643) -> (x .and. y?=w2644:bool)
            n851 = case shown="\"Start Task 1\", Default" w2645 {
              tunnel: w2644 -> [w2651 _]
              tunnel: [w2658 State_Type_Definitions,_for_0.26g_versions_and_later_2."True Stop" ("Enum")] -> w2640
              tunnel: w2634 -> [w2650 _]
              tunnel: w2638 -> [w2657 w2674]
              tunnel: [w2656 w2675] -> w2639
              tunnel: [State_Type_Definitions,_for_0.26g_versions_and_later_2."Idle" ("Enum") State_Type_Definitions,_for_0.26g_versions_and_later_2."Shutdown" ("Enum")] -> w2641
              frame "Start Task 1", Default {
                n852 = case shown="False" w2651 {
                  tunnel: w2657 -> [w2661 w2668]
                  tunnel: [w2662 w2667] -> w2656
                  frame False {
                    n853 = for {
                      tunnel: string[] ["READ LINE SENSOR", "READ NAVX", "RIGHT", "READ ENCODERS"] ("element") -> [w2663] mode=indexing
                      shift-right: [w2665] -> w2662
                      shift-left: w2661 -> [w2664]
                      n854 = Enqueue Element(queue=w2664, element=w2663) -> (queue out=w2665:refnum<queue>)  [unwired: 2 in, 2 out]
                    }
                  }
                  frame True {
                    n855 = for {
                      shift-right: [w2670] -> w2667
                      shift-left: w2668 -> [w2671]
                      tunnel: string[] ["STOP", "RESET ENCODERS", "RESET YAW", "OPEN LIFE CAM", "SET TIMER 2", "RESET FLAGS"] -> [w2669] mode=indexing
                      n856 = Enqueue Element(queue=w2671, element=w2669) -> (queue out=w2670:refnum<queue>)  [unwired: 2 in, 2 out]